vi "Velociprobe_Nanopositioner_Control_RT 2.vi"() -> ()   [LabVIEW 2015]
uses:
  <vilib>/rvi/interface/nirviReadWriteControl/nirviReadWriteControl.xnode
  <vilib>/rvi/interface/Simulation/niFpgaSimulationCallBeginRW.vi
  <vilib>/rvi/errors/niLvFpgaAdjustHostInterfaceError.vi
  <vilib>/rvi/interface/nirviCloseFPGA/nirviCloseFPGA.xnode
  <vilib>/rvi/interface/nirviMethod/nirviMethod.xnode
  <vilib>/rvi/errors/niLvFpgaMergeErrorWithErrorCode.vi
  <vilib>/Platform/TimedLoop/XDataNode/XDataNode.xnode
  <vilib>/Platform/TimedLoop/XDataNode/nitl_modes.ctl
  <vilib>/Platform/TimedLoop/XDataNode/XDNodeRunTimeDep.lvlib
  <vilib>/Platform/TimedLoop/XDataNode/wakeup.ctl
  <vilib>/Platform/TimedLoop/XDataNode/timing_clust.ctl
  <vilib>/rvi/interface/nirviOpenFPGA/nirviOpenFPGA.xnode
  <vilib>/rvi/Analysis/host/Public/NI_FpgaMspHost.lvlib
  State Enum.ctl
  Data Write Control.ctl
  <vilib>/rvi/interface/nirviMethod/StockFPGA_InlinedMethodWaitForSingleIRQ.vi
  <vilib>/FPGAPlugInAG/Dynamic/niLvFpga_WaitOnIrq_Dynamic.vi
  <vilib>/FPGAPlugInAG/Dynamic/niLvFpga_AcknowledgeIrq_Dynamic.vi
  <vilib>/Utility/file.llb/Read Delimited Spreadsheet (DBL).vi
  <vilib>/FPGAPlugInAG/Dynamic/niLvFpga_ConfigureFifo_Dynamic.vi
  NiFpgaLv.dll
  <vilib>/Utility/error.llb/Error Cluster From Error Code.vi
  <vilib>/FPGAPlugInAG/Dynamic/niLvFpga_ReadFifo_Dynamic.vi
  <vilib>/FPGAPlugInAG/Dynamic/niLvFpga_StopFifo_Dynamic.vi
  <vilib>/FPGAPlugInAG/Dynamic/niLvFpga_Close_Dynamic.vi
  FPGA Bitfiles/VelociprobeMIMOC_FPGATarget_VelociprobeNanop_-KB3D2agfK0.lvbitx
  FPGA VIs/Velociprobe_Nanopositioner_Control_FPGA.vi
  <vilib>/FPGAPlugInAG/cRIO-9039/niLvFpga_Open_cRIO-9039.vi
  <vilib>/rvi/interface/common/dynamic/niFpgaDynamicAddResources.vi
panel:
  in  "Tab Control":T1(tab)
  in  "Controller Time Period (uSec)":u32=40
  in  "Controller Output Time Period (uSec)":u32=40
  in  "X Reference Time Period (uSec)":u32=40
  in  "Plant Output Time Period (uSec)":u32=40
  in  "Stop":bool
  in  "Datalog Time Period (uSec)":u32=40
  in  "Analog Input Time Period (uSec)":u32=40
  in  "Detector Trigger Time Period (uSec)":u32=40
  in  "Trigger Generation Time Period (uSec)":u32=40
  in  "Y Reference Time Period (uSec)":u32=40
  in  "Z Reference Time Period (uSec)":u32=40
  in  "Data Trigger Time Period (uSec)":u32=40
  out "Iteration Duration RT Timed-Loop":i64=128
  in  "X Ramp Start (nm)":fxp<+/-,16,16>=-4500.0
  in  "X Ramp End (nm)":fxp<+/-,16,16>=4500.0
  in  "X Start Marker (nm)":fxp<+/-,58,25>
  in  "Y Ramp Start (nm)":fxp<+/-,16,16>=4500.0
  in  "Y Ramp End (nm)":fxp<+/-,16,16>=-4500.0
  in  "Y Vertical Step Size (nm)":fxp<+/-,16,16>=50.0
  in  "Y Start Marker (nm)":fxp<+/-,58,25>
  out "Fly Scan Running":bool
  out "Continue Run":bool
  out "X Ramp Period (usec)":fxp<+,24,24>=60000.0
  out "Y Ramp Period (usec)":fxp<+,24,24>=60000.0
  out "# of Hor Lines":fxp<+/-,34,18>=181.0 format="%.22g"
  in  "X Horizontal Step Size (nm)":fxp<+/-,16,16>=50.0
  out "# of Points per Line":fxp<+/-,33,17>=180.0
  out "# Total Trigger Points":fxp<+/-,64,34>=32580.0
  out "sec per line":dbl=0.06
  out "line per sec (Hz)":dbl=16.666666666666668
  out "X Ramp Period DBL (usec)":dbl=60000.0 format="%#_6f"
  out "Total Scan Time (sec)":dbl=10.86
  in  "Snake Scan Reference FPGA or EPICS":enum16{"FPGA Snake Scan", "EPICS Snake Scan"}(ring)
  in  "Detector Trigger Lower Limit (V)":fxp<+/-,20,5>
  in  "Detector Trigger Upper Limit (V)":fxp<+/-,20,5>=5.0
  out "Detector Trigger (V)":fxp<+/-,20,5>
  out "Detector Trigger In Range?":bool=TRUE
  in  "Trigger High Period (usec)":fxp<+/-,64,45>=1250.0
  in  "Trigger Low Period (usec)":fxp<+/-,64,45>=1250.0
  in  "Trigger High Level (V)":fxp<+/-,20,5>=5.0
  in  "Trigger Low Level (V)":fxp<+/-,20,5>
  in  "Trigger Wave Generator":T2(ring)=enum."Square Wave 1"
  in  "DT Reference Amplitude (V)":fxp<+/-,40,17>=5.0
  in  "DT Reference DC Offset (V)":fxp<+/-,16,16>
  out "DT Frequency (periods/tick)":fxp<+,32,0>=7.500010542571545e-05
  out "DT Phase Offset (periods)":fxp<+,32,0>
  in  "DT Reset":bool
  out "DT Duty Cycle (periods)":fxp<+,32,0>=0.8799999998882413
  in  "DT phase offset (deg)":dbl format="%#.6g"
  in  "DT Frequency (Hz)":dbl=3000.0 format="%#_6p"
  in  "DT duty cycle (%)":dbl=88.0 min=0.0 max=100.0 step=1.0
  in  "name":string="Velociprobe_Id_A344_.csv"
  in  "Write Data":bool
  in  "System Loop Type":enum16{"Open Loop", "Closed Loop"}(ring)=enum."Closed Loop"
  in  "Reset All":bool
  in  "Fly Scan Start":bool
  in  "Z White Noise Seed":u32=4
  in  "Z White Noise Amplitude":u16=32767
  in  "Y White Noise Seed":u32=4
  in  "Y White Noise Amplitude":u16=32767
  in  "Z Reference Reset":bool
  in  "Y Reference Reset":bool
  in  "X Reference Reset":bool
  in  "Z Reference Wave Selection":T3(ring)=enum."Sine Wave"
  in  "X Reference Wave Selection":T4(ring)=enum."Custom Up Down Ramp"
  in  "Y Reference Wave Selection":T5(ring)=enum."Custom Ramp Wave"
  in  "Optics and or Sample Stage":T6(ring)
  out "Z phase offset (periods)":fxp<+,32,0>
  out "Z frequency (periods/tick)":fxp<+,32,0>=1.25030055642128e-07 format="%.32g"
  in  "Z phase offset (deg)":dbl format="%#.6g"
  in  "Z frequency (Hz)":dbl=5.0 format="%#_6p"
  out "Y phase offset (periods)":fxp<+,32,0>
  out "Y frequency (periods/tick)":fxp<+,32,0>=5.005858838558197e-08 format="%.32g"
  in  "Y phase offset (deg)":dbl format="%#.6g"
  in  "Y frequency (Hz)":dbl=2.0 format="%#_6p"
  in  "Scaling mV to V":fxp<+,33,10>=0.001000046730041504
  out "Z Stage Reference (nm)":fxp<+/-,58,25>
  out "Y Stage Reference (nm)":fxp<+/-,58,25>
  out "X Stage Reference (nm)":fxp<+/-,58,25>
  in  "X White Noise Seed":u32=4
  in  "X White Noise Amplitude":u16=32767
  in  "Z Reference DC Offset (nm)":fxp<+/-,15,15>
  in  "Y Reference DC Offset (nm)":fxp<+/-,16,16>
  in  "X Reference DC Offset (nm)":fxp<+/-,16,16>
  in  "Z Reference Amplitude (nm)":fxp<+/-,40,17>
  in  "Y Reference Amplitude (nm)":fxp<+/-,40,17>=100.0
  in  "X Reference Amplitude (nm)":fxp<+/-,40,17>=100.0
  out "X phase offset (periods)":fxp<+,32,0>
  out "X frequency (periods/tick)":fxp<+,32,0>=1.25030055642128e-07 format="%.32g"
  in  "X phase offset (deg)":dbl format="%#.6g"
  in  "X frequency (Hz)":dbl=5.0 format="%#_6p"
  out "Trigger for Data":fxp<+/-,58,25>=1.0
  in  "Z-Stage Scaling Direction":fxp<+/-,3,3>=-1.0
  in  "Y-Stage Scaling Direction":fxp<+/-,3,3>=-1.0
  in  "Mod 3 AI2 V to nm Scaling":fxp<+,47,18>=1000.0
  in  "Mod 3 AI1 V to nm Scaling":fxp<+,47,18>=1000.0
  out "Mod6/DIO3":bool
  out "Mod5/DIO3":bool
  out "Mod4/DIO3":bool
  in  "Sample Z Stage Resolution (nm)":fxp<+,33,3>=0.5
  in  "Sample Y Stage Resolution (nm)":fxp<+,33,3>=0.5
  in  "Sample X Stage Resolution (nm)":fxp<+,33,3>=0.5
  in  "Optics Z Stage Resolution (nm)":fxp<+,33,3>=0.5
  in  "Optics Y Stage Resolution (nm)":fxp<+,33,3>=0.5
  in  "Optics X Stage Resolution (nm)":fxp<+,33,3>=0.5
  in  "Sample Z Reset":bool
  in  "Sample Y Reset":bool
  in  "Sample X Reset":bool
  out "Data":fxp<+/-,58,25>[](array[numeric])
  in  "Mod 3 AI0 V to nm Scaling":fxp<+,47,18>=1000.0
  in  "Timeout FPGA FIFO1":i32=40000000
  out "FIFO Timed Out":bool
  out "stop case":bool
  in  "IRQ Timeout (ms)":i32=10000
  out "IRQ Timed Out":bool
  in  "Datalog Cases":T7(ring)=enum."Data Log 16"
  out "Mod6/DIO2":bool
  out "Mod6/DIO1":bool
  out "Mod6/DIO0":bool=TRUE
  out "Mod5/DIO2":bool
  out "Mod5/DIO1":bool=TRUE
  out "Mod5/DIO0":bool
  out "Mod4/DIO2":bool=TRUE
  out "Mod4/DIO1":bool
  out "Mod4/DIO0":bool=TRUE
  in  "Optics Z Reset":bool
  in  "Optics Y Reset":bool
  in  "Optics X Reset":bool
  out "FIFO Timed Out?":bool
  in  "FIFO Time Period":dbl=0.01 format="%#_13g"
  out "Number of Elements":u32=1250
  out "Datalog Rate (Hz)":dbl=25000.000000000004
  out "Elements Remaining":u32
  in  "Timeout (ms)":i32=10000
  out "Number of Data Strings":i32=5
  out "Z-Stage Input In Range?":bool=TRUE
  out "Y-Stage Input In Range?":bool=TRUE
  out "X-Stage Input In Range?":bool=TRUE
  out "PI Z-Stage Input (V)":fxp<+/-,20,5>=-0.000732421875
  out "PI Y-Stage Input (V)":fxp<+/-,20,5>=0.005584716796875
  out "PI X-Stage Input (V)":fxp<+/-,20,5>=-0.00311279296875
  in  "Z-Stage nm to V Scaling":fxp<+/-,32,12>=0.0005397796630859375
  in  "Y-Stage nm to V Scaling":fxp<+/-,32,12>=0.0014200210571289062
  in  "X-Stage Scaling Direction":fxp<+/-,3,3>=-1.0
  in  "X-Stage nm to V Scaling":fxp<+/-,32,12>=0.0005359649658203125
  in  "Controller Output Lower Limit":fxp<+/-,20,5>=-5.0
  in  "Controller Output Upper Limit":fxp<+/-,20,5>=5.0
  out "Actual Depth":u32=131068416
  in  "Requested Depth":u32=131068000
  out "Waveform Graph 2":cluster{"t0":dbl, dbl, dbl[][]}(graph)={"t0"=0.0, 3.9999999999999996e-05, [[0.0, 0.0, 0.0, 0.0, 0.0, 0.0, 0.0, 0.0, 0.0, 0.0, 0.0, 0.0, 0.0, 0.0, 0.0, 0.0, 0.0, 0.0, 0.0, 0.0, 0.0, 0.0, 0.0, 0.0, 0.0, 0.0, 0.0, 0.0, 0.0, 0.0, 0.0, 0.0, 0.0, 0.0, 0.0, 0.0, 0.0, 0.0, 0.0, 0.0, 0.0, 0.0, 0.0, 0.0, 0.0, 0.0, 0.0, 0.0, 0.0, 0.0, 0.0, 0.0, 0.0, 0.0, 0.0, 0.0, 0.0, 0.0, 0.0, 0.0, 0.0, 0.0, 0.0, 0.0, 0.0, 0.0, 0.0, 0.0, 0.0, 0.0, 0.0, 0.0, 0.0, 0.0, 0.0, 0.0, 0.0, 0.0, 0.0, 0.0, 0.0, 0.0, 0.0, 0.0, 0.0, 0.0, 0.0, 0.0, 0.0, 0.0, 0.0, 0.0, 0.0, 0.0, 0.0, 0.0, 0.0, 0.0, 0.0, 0.0, 0.0, 0.0, 0.0, 0.0, 0.0, 0.0, 0.0, 0.0, 0.0, 0.0, 0.0, 0.0, 0.0, 0.0, 0.0, 0.0, 0.0, 0.0, 0.0, 0.0, 0.0, 0.0, 0.0, 0.0, 0.0, 0.0, 0.0, 0.0, 0.0, 0.0, 0.0, 0.0, 0.0, 0.0, 0.0, 0.0, 0.0, 0.0, 0.0, 0.0, 0.0, 0.0, 0.0, 0.0, 0.0, 0.0, 0.0, 0.0, 0.0, 0.0, 0.0, 0.0, 0.0, 0.0, 0.0, 0.0, 0.0, 0.0, 0.0, 0.0, 0.0, 0.0, 0.0, 0.0, 0.0, 0.0, 0.0, 0.0, 0.0, 0.0, 0.0, 0.0, 0.0, 0.0, 0.0, 0.0, 0.0, 0.0, 0.0, 0.0, 0.0, 0.0, 0.0, 0.0, 0.0, 0.0, 0.0, 0.0, 0.0, 0.0, 0.0, 0.0, 0.0, 0.0, 0.0, 0.0, 0.0, 0.0, 0.0, 0.0, 0.0, 0.0, 0.0, 0.0, 0.0, 0.0, 0.0, 0.0, 0.0, 0.0, 0.0, 0.0, 0.0, 0.0, 0.0, 0.0, 0.0, 0.0, 0.0, 0.0, 0.0, 0.0, 0.0, 0.0, 0.0, 0.0, 0.0, 0.0, 0.0, 0.0, 0.0, 0.0, 0.0, 0.0, 0.0, 0.0, 0.0, 0.0, 0.0, 0.0, 0.0, 0.0, 0.0, 0.0, 0.0, 0.0, 0.0, 0.0, 0.0, 0.0], [0.0, 0.0, 0.0, 0.0, 0.0, 0.0, 0.0, 0.0, 0.0, 0.0, 0.0, 0.0, 0.0, 0.0, 0.0, 0.0, 0.0, 0.0, 0.0, 0.0, 0.0, 0.0, 0.0, 0.0, 0.0, 0.0, 0.0, 0.0, 0.0, 0.0, 0.0, 0.0, 0.0, 0.0, 0.0, 0.0, 0.0, 0.0, 0.0, 0.0, 0.0, 0.0, 0.0, 0.0, 0.0, 0.0, 0.0, 0.0, 0.0, 0.0, 0.0, 0.0, 0.0, 0.0, 0.0, 0.0, 0.0, 0.0, 0.0, 0.0, 0.0, 0.0, 0.0, 0.0, 0.0, 0.0, 0.0, 0.0, 0.0, 0.0, 0.0, 0.0, 0.0, 0.0, 0.0, 0.0, 0.0, 0.0, 0.0, 0.0, 0.0, 0.0, 0.0, 0.0, 0.0, 0.0, 0.0, 0.0, 0.0, 0.0, 0.0, 0.0, 0.0, 0.0, 0.0, 0.0, 0.0, 0.0, 0.0, 0.0, 0.0, 0.0, 0.0, 0.0, 0.0, 0.0, 0.0, 0.0, 0.0, 0.0, 0.0, 0.0, 0.0, 0.0, 0.0, 0.0, 0.0, 0.0, 0.0, 0.0, 0.0, 0.0, 0.0, 0.0, 0.0, 0.0, 0.0, 0.0, 0.0, 0.0, 0.0, 0.0, 0.0, 0.0, 0.0, 0.0, 0.0, 0.0, 0.0, 0.0, 0.0, 0.0, 0.0, 0.0, 0.0, 0.0, 0.0, 0.0, 0.0, 0.0, 0.0, 0.0, 0.0, 0.0, 0.0, 0.0, 0.0, 0.0, 0.0, 0.0, 0.0, 0.0, 0.0, 0.0, 0.0, 0.0, 0.0, 0.0, 0.0, 0.0, 0.0, 0.0, 0.0, 0.0, 0.0, 0.0, 0.0, 0.0, 0.0, 0.0, 0.0, 0.0, 0.0, 0.0, 0.0, 0.0, 0.0, 0.0, 0.0, 0.0, 0.0, 0.0, 0.0, 0.0, 0.0, 0.0, 0.0, 0.0, 0.0, 0.0, 0.0, 0.0, 0.0, 0.0, 0.0, 0.0, 0.0, 0.0, 0.0, 0.0, 0.0, 0.0, 0.0, 0.0, 0.0, 0.0, 0.0, 0.0, 0.0, 0.0, 0.0, 0.0, 0.0, 0.0, 0.0, 0.0, 0.0, 0.0, 0.0, 0.0, 0.0, 0.0, 0.0, 0.0, 0.0, 0.0, 0.0, 0.0, 0.0, 0.0, 0.0, 0.0, 0.0, 0.0, 0.0, 0.0, 0.0, 0.0, 0.0, 0.0], [0.0, 0.0, 0.0, 0.0, 0.0, 0.0, 0.0, 0.0, 0.0, 0.0, 0.0, 0.0, 0.0, 0.0, 0.0, 0.0, 0.0, 0.0, 0.0, 0.0, 0.0, 0.0, 0.0, 0.0, 0.0, 0.0, 0.0, 0.0, 0.0, 0.0, 0.0, 0.0, 0.0, 0.0, 0.0, 0.0, 0.0, 0.0, 0.0, 0.0, 0.0, 0.0, 0.0, 0.0, 0.0, 0.0, 0.0, 0.0, 0.0, 0.0, 0.0, 0.0, 0.0, 0.0, 0.0, 0.0, 0.0, 0.0, 0.0, 0.0, 0.0, 0.0, 0.0, 0.0, 0.0, 0.0, 0.0, 0.0, 0.0, 0.0, 0.0, 0.0, 0.0, 0.0, 0.0, 0.0, 0.0, 0.0, 0.0, 0.0, 0.0, 0.0, 0.0, 0.0, 0.0, 0.0, 0.0, 0.0, 0.0, 0.0, 0.0, 0.0, 0.0, 0.0, 0.0, 0.0, 0.0, 0.0, 0.0, 0.0, 0.0, 0.0, 0.0, 0.0, 0.0, 0.0, 0.0, 0.0, 0.0, 0.0, 0.0, 0.0, 0.0, 0.0, 0.0, 0.0, 0.0, 0.0, 0.0, 0.0, 0.0, 0.0, 0.0, 0.0, 0.0, 0.0, 0.0, 0.0, 0.0, 0.0, 0.0, 0.0, 0.0, 0.0, 0.0, 0.0, 0.0, 0.0, 0.0, 0.0, 0.0, 0.0, 0.0, 0.0, 0.0, 0.0, 0.0, 0.0, 0.0, 0.0, 0.0, 0.0, 0.0, 0.0, 0.0, 0.0, 0.0, 0.0, 0.0, 0.0, 0.0, 0.0, 0.0, 0.0, 0.0, 0.0, 0.0, 0.0, 0.0, 0.0, 0.0, 0.0, 0.0, 0.0, 0.0, 0.0, 0.0, 0.0, 0.0, 0.0, 0.0, 0.0, 0.0, 0.0, 0.0, 0.0, 0.0, 0.0, 0.0, 0.0, 0.0, 0.0, 0.0, 0.0, 0.0, 0.0, 0.0, 0.0, 0.0, 0.0, 0.0, 0.0, 0.0, 0.0, 0.0, 0.0, 0.0, 0.0, 0.0, 0.0, 0.0, 0.0, 0.0, 0.0, 0.0, 0.0, 0.0, 0.0, 0.0, 0.0, 0.0, 0.0, 0.0, 0.0, 0.0, 0.0, 0.0, 0.0, 0.0, 0.0, 0.0, 0.0, 0.0, 0.0, 0.0, 0.0, 0.0, 0.0, 0.0, 0.0, 0.0, 0.0, 0.0, 0.0, 0.0, 0.0, 0.0, 0.0, 0.0, 0.0], [0.0, 0.0, 0.0, 0.0, 0.0, 0.0, 0.0, 0.0, 0.0, 0.0, 0.0, 0.0, 0.0, 0.0, 0.0, 0.0, 0.0, 0.0, 0.0, 0.0, 0.0, 0.0, 0.0, 0.0, 0.0, 0.0, 0.0, 0.0, 0.0, 0.0, 0.0, 0.0, 0.0, 0.0, 0.0, 0.0, 0.0, 0.0, 0.0, 0.0, 0.0, 0.0, 0.0, 0.0, 0.0, 0.0, 0.0, 0.0, 0.0, 0.0, 0.0, 0.0, 0.0, 0.0, 0.0, 0.0, 0.0, 0.0, 0.0, 0.0, 0.0, 0.0, 0.0, 0.0, 0.0, 0.0, 0.0, 0.0, 0.0, 0.0, 0.0, 0.0, 0.0, 0.0, 0.0, 0.0, 0.0, 0.0, 0.0, 0.0, 0.0, 0.0, 0.0, 0.0, 0.0, 0.0, 0.0, 0.0, 0.0, 0.0, 0.0, 0.0, 0.0, 0.0, 0.0, 0.0, 0.0, 0.0, 0.0, 0.0, 0.0, 0.0, 0.0, 0.0, 0.0, 0.0, 0.0, 0.0, 0.0, 0.0, 0.0, 0.0, 0.0, 0.0, 0.0, 0.0, 0.0, 0.0, 0.0, 0.0, 0.0, 0.0, 0.0, 0.0, 0.0, 0.0, 0.0, 0.0, 0.0, 0.0, 0.0, 0.0, 0.0, 0.0, 0.0, 0.0, 0.0, 0.0, 0.0, 0.0, 0.0, 0.0, 0.0, 0.0, 0.0, 0.0, 0.0, 0.0, 0.0, 0.0, 0.0, 0.0, 0.0, 0.0, 0.0, 0.0, 0.0, 0.0, 0.0, 0.0, 0.0, 0.0, 0.0, 0.0, 0.0, 0.0, 0.0, 0.0, 0.0, 0.0, 0.0, 0.0, 0.0, 0.0, 0.0, 0.0, 0.0, 0.0, 0.0, 0.0, 0.0, 0.0, 0.0, 0.0, 0.0, 0.0, 0.0, 0.0, 0.0, 0.0, 0.0, 0.0, 0.0, 0.0, 0.0, 0.0, 0.0, 0.0, 0.0, 0.0, 0.0, 0.0, 0.0, 0.0, 0.0, 0.0, 0.0, 0.0, 0.0, 0.0, 0.0, 0.0, 0.0, 0.0, 0.0, 0.0, 0.0, 0.0, 0.0, 0.0, 0.0, 0.0, 0.0, 0.0, 0.0, 0.0, 0.0, 0.0, 0.0, 0.0, 0.0, 0.0, 0.0, 0.0, 0.0, 0.0, 0.0, 0.0, 0.0, 0.0, 0.0, 0.0, 0.0, 0.0, 0.0, 0.0, 0.0, 0.0, 0.0, 0.0], [0.0, 0.0, 0.0, 0.0, 0.0, 0.0, 0.0, 0.0, 0.0, 0.0, 0.0, 0.0, 0.0, 0.0, 0.0, 0.0, 0.0, 0.0, 0.0, 0.0, 0.0, 0.0, 0.0, 0.0, 0.0, 0.0, 0.0, 0.0, 0.0, 0.0, 0.0, 0.0, 0.0, 0.0, 0.0, 0.0, 0.0, 0.0, 0.0, 0.0, 0.0, 0.0, 0.0, 0.0, 0.0, 0.0, 0.0, 0.0, 0.0, 0.0, 0.0, 0.0, 0.0, 0.0, 0.0, 0.0, 0.0, 0.0, 0.0, 0.0, 0.0, 0.0, 0.0, 0.0, 0.0, 0.0, 0.0, 0.0, 0.0, 0.0, 0.0, 0.0, 0.0, 0.0, 0.0, 0.0, 0.0, 0.0, 0.0, 0.0, 0.0, 0.0, 0.0, 0.0, 0.0, 0.0, 0.0, 0.0, 0.0, 0.0, 0.0, 0.0, 0.0, 0.0, 0.0, 0.0, 0.0, 0.0, 0.0, 0.0, 0.0, 0.0, 0.0, 0.0, 0.0, 0.0, 0.0, 0.0, 0.0, 0.0, 0.0, 0.0, 0.0, 0.0, 0.0, 0.0, 0.0, 0.0, 0.0, 0.0, 0.0, 0.0, 0.0, 0.0, 0.0, 0.0, 0.0, 0.0, 0.0, 0.0, 0.0, 0.0, 0.0, 0.0, 0.0, 0.0, 0.0, 0.0, 0.0, 0.0, 0.0, 0.0, 0.0, 0.0, 0.0, 0.0, 0.0, 0.0, 0.0, 0.0, 0.0, 0.0, 0.0, 0.0, 0.0, 0.0, 0.0, 0.0, 0.0, 0.0, 0.0, 0.0, 0.0, 0.0, 0.0, 0.0, 0.0, 0.0, 0.0, 0.0, 0.0, 0.0, 0.0, 0.0, 0.0, 0.0, 0.0, 0.0, 0.0, 0.0, 0.0, 0.0, 0.0, 0.0, 0.0, 0.0, 0.0, 0.0, 0.0, 0.0, 0.0, 0.0, 0.0, 0.0, 0.0, 0.0, 0.0, 0.0, 0.0, 0.0, 0.0, 0.0, 0.0, 0.0, 0.0, 0.0, 0.0, 0.0, 0.0, 0.0, 0.0, 0.0, 0.0, 0.0, 0.0, 0.0, 0.0, 0.0, 0.0, 0.0, 0.0, 0.0, 0.0, 0.0, 0.0, 0.0, 0.0, 0.0, 0.0, 0.0, 0.0, 0.0, 0.0, 0.0, 0.0, 0.0, 0.0, 0.0, 0.0, 0.0, 0.0, 0.0, 0.0, 0.0, 0.0, 0.0, 0.0, 0.0, 0.0, 0.0]]}
  out "Elements Remaining Waveform Chart":u32(graph)
  out "Elements Remaining Waveform Chart 3":u32(graph)
  out "XY Graph":cluster{"Array":dbl[], "Array":dbl[]}(graph)
  out "XY Graph 2":cluster{"Array":dbl[], "Array":dbl[]}(graph)
  out "Measured Datalog Time Period (Ticks)":u32=1600
  out "Measured Datalog Loop Rate (secs)":dbl=3.9999999999999996e-05
  out "Measured Datalog Loop Rate (kHz)":dbl=25.000000000000004
  out "Measured Counter Loop Rate (secs)":dbl
  out "Measured Counter Loop Rate (MHz)":dbl=inf
  out "Measured X Reference Loop Rate (secs)":dbl=3.9999999999999996e-05
  out "Measured X Reference Loop Rate (kHz)":dbl=25.000000000000004
  out "Measured X Reference Time Period (Ticks)":u32=1600
  out "Measured Controller Loop Rate (kHz)":dbl=25.000000000000004
  out "Measured Controller Output Loop Rate (secs)":dbl=3.9999999999999996e-05
  out "Measured Controller Output Loop Rate (kHz)":dbl=25.000000000000004
  out "Measured Plant Output Loop Rate (secs)":dbl=3.9999999999999996e-05
  out "Measured Plant Output Loop Rate (kHz)":dbl=25.000000000000004
  out "Measured Controller Loop Rate (secs)":dbl=3.9999999999999996e-05
  out "Measured Controller Time Period (Ticks)":u32=1600
  out "Datalog Time Period (sec)":dbl=3.9999999999999996e-05
  out "Measured Controller Output Time Period (Ticks)":u32=1600
  out "Measured Plant Output Time Period (Ticks)":u32=1600
  out "Measured Counter Time Period (Ticks)":u32
  out "32 bit Count Optics X":i32
  out "32 bit Count Optics  Y":i32
  out "32 bit Count Optics  Z":i32
  out "32 bit Count Sample X":i32
  out "32 bit Count Sample  Y":i32=2
  out "32 bit Count Sample  Z":i32=-4
  out "Optics X Stage Displacement (nm)":fxp<+/-,58,25>=-1.0
  out "Optics Y Stage Displacement (nm)":fxp<+/-,58,25>
  out "Optics Z Stage Displacement (nm)":fxp<+/-,58,25>
  out "Sample X Stage Displacement (nm)":fxp<+/-,58,25>=-0.5
  out "Sample Y Stage Displacement (nm)":fxp<+/-,58,25>=1.5
  out "Sample Z Stage Displacement (nm)":fxp<+/-,58,25>=-1.0
  out "Measured Analog Input Time Period (Ticks)":u32=1600
  out "Measured Analog Input Loop Rate (secs)":dbl=3.9999999999999996e-05
  out "Measured Analog Input Loop Rate (kHz)":dbl=25.000000000000004
  out "Measured Detector Trigger Time Period (Ticks)":u32=1600
  out "Measured Trigger Gen Time Period (Ticks)":u32=1600
  out "Measured Y Reference Time Period (Ticks)":u32=1600
  out "Measured Z Reference Time Period (Ticks)":u32=1600
  out "Measured Y Reference Loop Rate (secs)":dbl=3.9999999999999996e-05
  out "Measured Y Reference Loop Rate (kHz)":dbl=25.000000000000004
  out "Measured Z Reference Loop Rate (secs)":dbl=3.9999999999999996e-05
  out "Measured Z Reference Loop Rate (kHz)":dbl=25.000000000000004
  out "Measured Data Trigger Time Period (Ticks)":u32=1600
  out "message":string="No Error"
  out "2iddVELO:VP:X_End_nm":dbl=2000.0
  out "2iddVELO:VP:X_Start_nm":dbl=-2000.0
  out "2iddVELO:VP:Flyscan_Start":bool
  out "2iddVELO:VP:Y_Start_nm":dbl=2000.0
  out "2iddVELO:VP:Y_End_nm":dbl=-2000.0
  out "2iddVELO:VP:Y_Step_Size_nm":dbl=50.0
  out "2iddVELO:VP:X_Step_Size_nm":dbl=50.0
  out "2iddVELO:VP:Trigger_Freq_Hz":dbl=1000.0
  out "2iddVELO:VP:Write_Data":bool
  out "2iddVELO:VP:Trig_DutyCycle_Per":dbl=99.0
  in  "file path soscoeff_xx1":path=path "C:/ni-rt/startup/2 ID D/Kxx/Kxx_1_Gxx_md_40us/Kxx_1_Gxx_matched_dow_16ord_mVpnm_cd8a3_AvTio9_X5nm_500pm_all_40us_soscof_xx1.mat"
  in  "file path sos gain SF Controller_xx1":path=path "C:/ni-rt/startup/2 ID D/Kxx/Kxx_1_Gxx_md_40us/Kxx_1_Gxx_matched_dow_16ord_mVpnm_cd8a3_AvTio9_X5nm_500pm_all_40us_soscof_xx2.mat"
  in  "file path soscoeff_yy1":path=path "C:/ni-rt/startup/2 ID D/Kyy/Kyy_trial_1_Gyy_md_40us/Kyy_trial_1_Gyy_matched_dow_8ord_mVpnm_cd8a3_AvTio9_Y5nm_500pm_all_40us_soscof_yy1.mat"
  in  "file path sos gain SF Controller_yy1":path=path "C:/ni-rt/startup/2 ID D/Kyy/Kyy_trial_1_Gyy_md_40us/Kyy_trial_1_Gyy_matched_dow_8ord_mVpnm_cd8a3_AvTio9_Y5nm_500pm_all_40us_soscof_yy2.mat"
  in  "file path soscoeff_zz1":path=path "C:/ni-rt/startup/2 ID D/Kzz/Kzz_1_Gzz_md_40us/Kzz_1_Gzz_matched_dow_29ord_mVpnm_cd8a3_AvTio9_Z5nm_500pm_all_40us_soscof_zz1.mat"
  in  "file path sos gain SF Controller_zz1":path=path "C:/ni-rt/startup/2 ID D/Kzz/Kzz_1_Gzz_md_40us/Kzz_1_Gzz_matched_dow_29ord_mVpnm_cd8a3_AvTio9_Z5nm_500pm_all_40us_soscof_zz2.mat"
  in  "file path soscoeff_yx1":path=path "C:/ni-rt/startup/2 ID D/Kxx/Kxx_1_Gxx_md_40us/allzero_mVpnm_XX_XY_XZ_YX_YY_YZ_ZX_ZY_ZZ_woffst_soscoeff1.mat"
  in  "file path sos gain SF Controller_yx1":path=path "C:/ni-rt/startup/2 ID D/Kxx/Kxx_1_Gxx_md_40us/allzero_mVpnm_XX_XY_XZ_YX_YY_YZ_ZX_ZY_ZZ_woffst_soscoeff2.mat"
  in  "file path soscoeff_zx1":path=path "C:/ni-rt/startup/2 ID D/Kxx/Kxx_1_Gxx_md_40us/allzero_mVpnm_XX_XY_XZ_YX_YY_YZ_ZX_ZY_ZZ_woffst_soscoeff1.mat"
  in  "file path sos gain SF Controller_zx1":path=path "C:/ni-rt/startup/2 ID D/Kxx/Kxx_1_Gxx_md_40us/allzero_mVpnm_XX_XY_XZ_YX_YY_YZ_ZX_ZY_ZZ_woffst_soscoeff2.mat"
  in  "file path soscoeff_xy1":path=path "C:/ni-rt/startup/2 ID D/Kxx/Kxx_1_Gxx_md_40us/allzero_mVpnm_XX_XY_XZ_YX_YY_YZ_ZX_ZY_ZZ_woffst_soscoeff1.mat"
  in  "file path sos gain SF Controller_xy1":path=path "C:/ni-rt/startup/2 ID D/Kxx/Kxx_1_Gxx_md_40us/allzero_mVpnm_XX_XY_XZ_YX_YY_YZ_ZX_ZY_ZZ_woffst_soscoeff2.mat"
  in  "file path soscoeff_zy1":path=path "C:/ni-rt/startup/2 ID D/Kxx/Kxx_1_Gxx_md_40us/allzero_mVpnm_XX_XY_XZ_YX_YY_YZ_ZX_ZY_ZZ_woffst_soscoeff1.mat"
  in  "file path sos gain SF Controller_zy1":path=path "C:/ni-rt/startup/2 ID D/Kxx/Kxx_1_Gxx_md_40us/allzero_mVpnm_XX_XY_XZ_YX_YY_YZ_ZX_ZY_ZZ_woffst_soscoeff2.mat"
  in  "file path soscoeff_xz1":path=path "C:/ni-rt/startup/2 ID D/Kxx/Kxx_1_Gxx_md_40us/allzero_mVpnm_XX_XY_XZ_YX_YY_YZ_ZX_ZY_ZZ_woffst_soscoeff1.mat"
  in  "file path sos gain SF Controller_xz1":path=path "C:/ni-rt/startup/2 ID D/Kxx/Kxx_1_Gxx_md_40us/allzero_mVpnm_XX_XY_XZ_YX_YY_YZ_ZX_ZY_ZZ_woffst_soscoeff2.mat"
  in  "file path soscoeff_yz1":path=path "C:/ni-rt/startup/2 ID D/Kxx/Kxx_1_Gxx_md_40us/allzero_mVpnm_XX_XY_XZ_YX_YY_YZ_ZX_ZY_ZZ_woffst_soscoeff1.mat"
  in  "file path sos gain SF Controller_yz1":path=path "C:/ni-rt/startup/2 ID D/Kxx/Kxx_1_Gxx_md_40us/allzero_mVpnm_XX_XY_XZ_YX_YY_YZ_ZX_ZY_ZZ_woffst_soscoeff2.mat"
  out "-a01(2) xx1c":fxp<+/-,64,9>[](array[numeric])=[0.637785025840232, 0.9924182654286198, 1.8461027816316544, 0.8635404845716299, 1.0670555456779864, 1.6350703383821101, 1.6323955588345012, 1.1102241390539636, 0.0, 0.0, 0.0, 0.0, 0.0, 0.0, 0.0, 0.0, 0.0, 0.0, 0.0, 0.0]
  out "-a02(2) xx1c":fxp<+/-,64,9>[](array[numeric])=[-0.999855815746439, -0.9676991072632725, -0.9642268720534838, -0.9446498323360957, -0.9442808087139987, -0.7547983908829242, -0.6690016013017409, -0.11027986125857198, 0.0, 0.0, 0.0, 0.0, 0.0, 0.0, 0.0, 0.0, 0.0, 0.0, 0.0, 0.0]
  out "b01(2) xx1c":fxp<+/-,64,9>[](array[numeric])=[-0.6378105164532328, -1.0062332697665268, -1.8762916543815855, -0.8616288879491845, -1.0856571140792324, -1.6862585929720944, -1.743591709663851, -0.6129835805090948, 0.0, 0.0, 0.0, 0.0, 0.0, 0.0, 0.0, 0.0, 0.0, 0.0, 0.0, 0.0]
  out "b02(2) xx1c":fxp<+/-,64,9>[](array[numeric])=[0.9999102047610771, 0.9971375605901365, 0.9926840301018772, 0.9509648854364836, 0.9563369558920378, 0.7818900462139817, 0.7642575436257291, 3.0531133177191805e-16, 0.0, 0.0, 0.0, 0.0, 0.0, 0.0, 0.0, 0.0, 0.0, 0.0, 0.0, 0.0]
  out "sos gain SF Controller xx1c":fxp<+/-,42,9>=-0.1625035791657865
  out "-a01(2) yy1c":fxp<+/-,64,9>[](array[numeric])=[1.8740229377643998, 1.3096977339382483, 1.7453886241944765, 0.2668895009727739, 0.0, 0.0, 0.0, 0.0, 0.0, 0.0, 0.0, 0.0, 0.0, 0.0, 0.0, 0.0, 0.0, 0.0, 0.0, 0.0]
  out "-a02(2) yy1c":fxp<+/-,64,9>[](array[numeric])=[-0.9732703278433918, -0.5194903821190732, -0.7453924481836136, -2.7755575615628914e-17, 0.0, 0.0, 0.0, 0.0, 0.0, 0.0, 0.0, 0.0, 0.0, 0.0, 0.0, 0.0, 0.0, 0.0, 0.0, 0.0]
  out "b01(2) yy1c":fxp<+/-,64,9>[](array[numeric])=[-1.8979173162254057, -1.8463149313261074, -1.7151162246453355, -0.006444279582847878, 0.0, 0.0, 0.0, 0.0, 0.0, 0.0, 0.0, 0.0, 0.0, 0.0, 0.0, 0.0, 0.0, 0.0, 0.0, 0.0]
  out "b02(2) yy1c":fxp<+/-,64,9>[](array[numeric])=[0.9969084979865663, 0.9421233904433339, 0.7362048104846675, 0.0, 0.0, 0.0, 0.0, 0.0, 0.0, 0.0, 0.0, 0.0, 0.0, 0.0, 0.0, 0.0, 0.0, 0.0, 0.0, 0.0]
  out "sos gain SF Controller yy1c":fxp<+/-,42,9>=-1.480983349494636
  out "-a01(2) zz1c":fxp<+/-,64,9>[](array[numeric])=[0.6242394224317618, 1.8967038692417004, 0.6659160318030806, 1.7792660019034106, 1.6870099721477447, 0.6417945190222861, 1.4838029149808185, 1.8456549628851837, 1.2189509782386598, 0.9933314517253298, 1.0158915520299678, 0.8863484387433826, 0.026837806879254994, 1.8269783715122585, 0.22448441435364225, 0.0, 0.0, 0.0, 0.0, 0.0]
  out "-a02(2) zz1c":fxp<+/-,64,9>[](array[numeric])=[-0.9983298461163967, -0.9972287452752734, -0.995744457243837, -0.9947210838396919, -0.9925914602095722, -0.9920974045271405, -0.9881915357970101, -0.9800069383591395, -0.9760641145386646, -0.9508624135515895, -0.9242774595356998, -0.655945641403593, -0.008661844724279444, -0.8269827070369743, 0.0, 0.0, 0.0, 0.0, 0.0, 0.0]
  out "b01(2) zz1c":fxp<+/-,64,9>[](array[numeric])=[-0.6245671059510156, -1.897930093390194, -0.6670970070931089, -1.7670265604573054, -1.6833314913922348, -0.6327437892303018, -1.5025901530730128, -1.8636454269915796, -1.1210694827766767, -0.9982206064398196, -1.0326369335418408, -1.1342635673267367, -1.6852506306166828, -0.9843740162364313, -1.7208456881689926e-15, 0.0, 0.0, 0.0, 0.0, 0.0]
  out "b02(2) zz1c":fxp<+/-,64,9>[](array[numeric])=[0.9973135069419645, 0.9951302056171929, 0.9993435624612031, 0.9919371251860779, 0.994931751453586, 0.9881092761723503, 0.9884874399279107, 0.9977145546300196, 0.9725302934743221, 0.9855561672767964, 0.9893454712398023, 0.846212786518208, 0.7855598927779743, 0.0978075435519738, 0.0, 0.0, 0.0, 0.0, 0.0, 0.0]
  out "sos gain SF Controller zz1c":fxp<+/-,42,9>=-0.1988595259608701
  out "-a01(2) yx1c":fxp<+/-,64,9>[](array[numeric])
  out "-a02(2) yx1c":fxp<+/-,64,9>[](array[numeric])
  out "b01(2) yx1c":fxp<+/-,64,9>[](array[numeric])
  out "b02(2) yx1c":fxp<+/-,64,9>[](array[numeric])
  out "sos gain SF Controller yx1c":fxp<+/-,42,9>
  out "-a01(2) zx1c":fxp<+/-,64,9>[](array[numeric])
  out "-a02(2) zx1c":fxp<+/-,64,9>[](array[numeric])
  out "b01(2) zx1c":fxp<+/-,64,9>[](array[numeric])
  out "b02(2) zx1c":fxp<+/-,64,9>[](array[numeric])
  out "sos gain SF Controller zx1c":fxp<+/-,42,9>
  out "-a01(2) xy1c":fxp<+/-,64,9>[](array[numeric])
  out "-a02(2) xy1c":fxp<+/-,64,9>[](array[numeric])
  out "b01(2) xy1c":fxp<+/-,64,9>[](array[numeric])
  out "b02(2) xy1c":fxp<+/-,64,9>[](array[numeric])
  out "sos gain SF Controller xy1c":fxp<+/-,42,9>
  out "-a01(2) zy1c":fxp<+/-,64,9>[](array[numeric])
  out "-a02(2) zy1c":fxp<+/-,64,9>[](array[numeric])
  out "b01(2) zy1c":fxp<+/-,64,9>[](array[numeric])
  out "b02(2) zy1c":fxp<+/-,64,9>[](array[numeric])
  out "sos gain SF Controller zy1c":fxp<+/-,42,9>
  out "-a01(2) xz1c":fxp<+/-,64,9>[](array[numeric])
  out "-a02(2) xz1c":fxp<+/-,64,9>[](array[numeric])
  out "b01(2) xz1c":fxp<+/-,64,9>[](array[numeric])
  out "b02(2) xz1c":fxp<+/-,64,9>[](array[numeric])
  out "sos gain SF Controller xz1c":fxp<+/-,42,9>
  out "-a01(2) yz1c":fxp<+/-,64,9>[](array[numeric])
  out "-a02(2) yz1c":fxp<+/-,64,9>[](array[numeric])
  out "b01(2) yz1c":fxp<+/-,64,9>[](array[numeric])
  out "b02(2) yz1c":fxp<+/-,64,9>[](array[numeric])
  out "sos gain SF Controller yz1c":fxp<+/-,42,9>
  out "error out (Sig Gen)":errorcluster
  out "error out (FPGA)":errorcluster
  out "error out (AO FPGA)":errorcluster
  out "Error (RT)":errorcluster
  out "error out (Sig Gen) 2":errorcluster
  out "error out (Sig Gen) 3":errorcluster
  out "error out (Sig Gen) 4":errorcluster
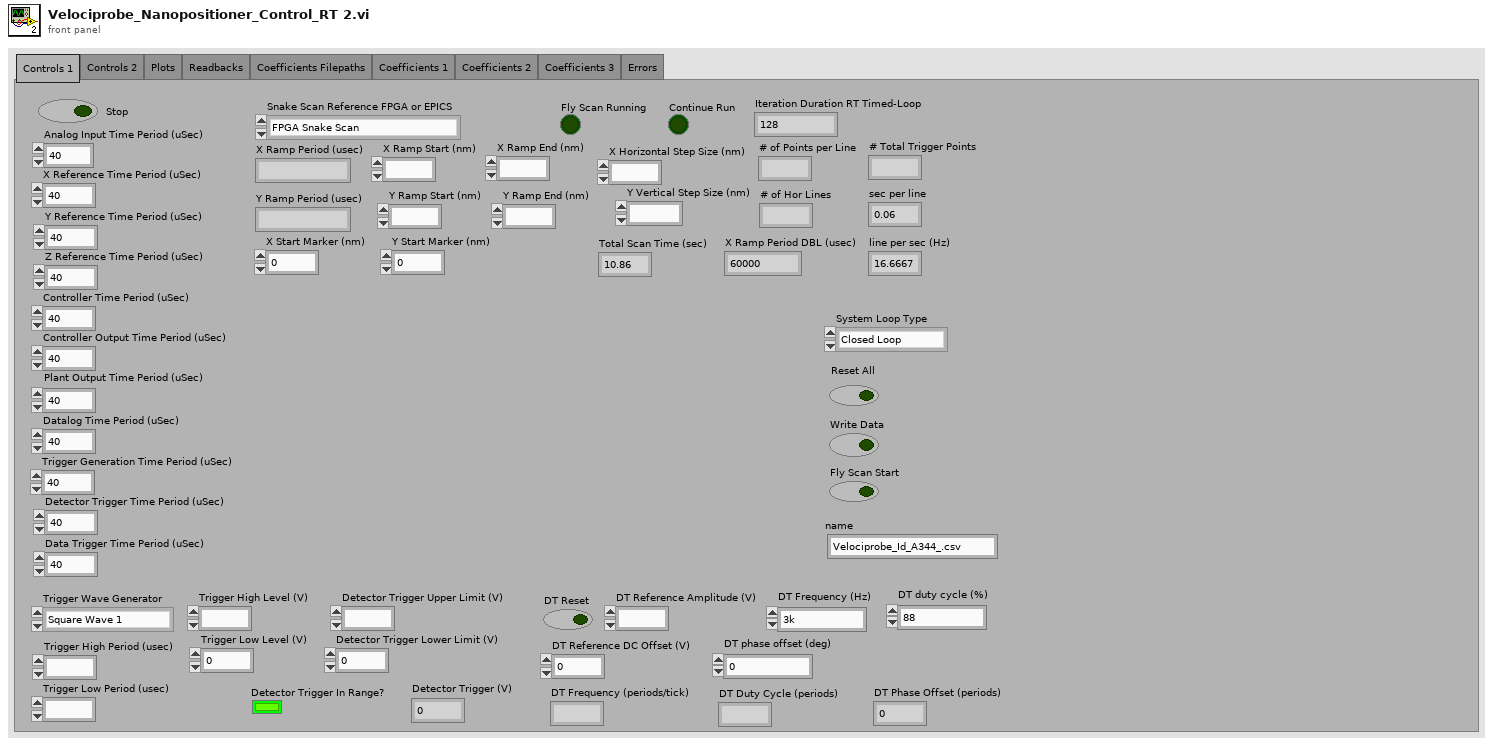
[diagram p1: front panel]
types:
  T1 = enum32{"Controls 1", "Controls 2", "Plots", "Readbacks", "Coefficients Filepaths", "Coefficients 1", "Coefficients 2", "Coefficients 3", "Errors"}
  T2 = enum16{"Custom Square Wave ", "Square Wave 1", "Square Wave 2"}
  T3 = enum16{"Constant", "Sine Wave", "Sawtooth Wave", "Square Wave", "Filtered White Noise"}
  T4 = enum16{"Constant", "Sine Wave", "Custom Up Down Ramp", "Filtered White Noise"}
  T5 = enum16{"Constant", "Sine Wave", "Custom Ramp Wave", "Filtered White Noise"}
  T6 = enum16{"Optics Stage Only", "Optics and Sample Stage"}
  T7 = enum16{"Data Log 1", "Data Log 2", "Data Log 3", "Data Log 4", "Data Log 5", "Data Log 6", "Data Log 7", "Data Log 8", "Data Log 9", "Data Log 10", "Data Log 11", "Data Log 12", "Data Log 13", "Data Log 14", "Data Log 15", "Data Log 16"}
  T8 = typedef "State Enum.ctl" = enum16{"Initialization", "Update Controller Info", "Update Reference Info", "Update Detector Trigger Info", "Update Datalog Info", "Check FPGA Status", "Reading FIFO", "Exit"}
  T9 = typedef "XDNodeRunTimeDep.lvlib/timing_clust.ctl" = cluster{"Expected End [f-1]":u64, "Actual End [f-1]":u64, "Finished Late? [f-1]":bool, "Expected End [i-1]":u64, "Actual End [i-1]":u64, "Finished Late? [i-1]":bool, "Expected Start [i]":u64, "Actual Start [i]":u64, "Expected Start [f]":u64, "Actual Start [f]":u64, "Source Name":string, "Structure Name":string, "Period":i64, "Deadline":i64, "Offset":i64, "Start":i64, "Priority":i32, "Timeout":i32, "Mode":T10, "Wakeup Reason":T11, "Error":errorcluster, "Source Type":string, "Secondary Source Type":string, "Global End Time":u64, "Global Start Time":u64, "Frame Duration":u64, "Iteration Duration":u64, "Assigned CPU":i32, "I/O Scan Engine Mode":u32}
  T10 = typedef "XDNodeRunTimeDep.lvlib/nitl_modes.ctl" = enum32{"No Change", "Process missed periods, maintain original phase", "Discard missed periods, maintain original phase", "Process missed periods, ignore original phase", "Discard missed periods, ignore original phase"}
  T11 = typedef "XDNodeRunTimeDep.lvlib/wakeup.ctl" = enum32{"Normal", "Aborted", "Asynchronous wakeup", "Timing source error", "Timed loop error", "Timeout"}
  T12 = typedef "Data Write Control.ctl" = enum16{"Initialize", "Read", "Write", "Close"}
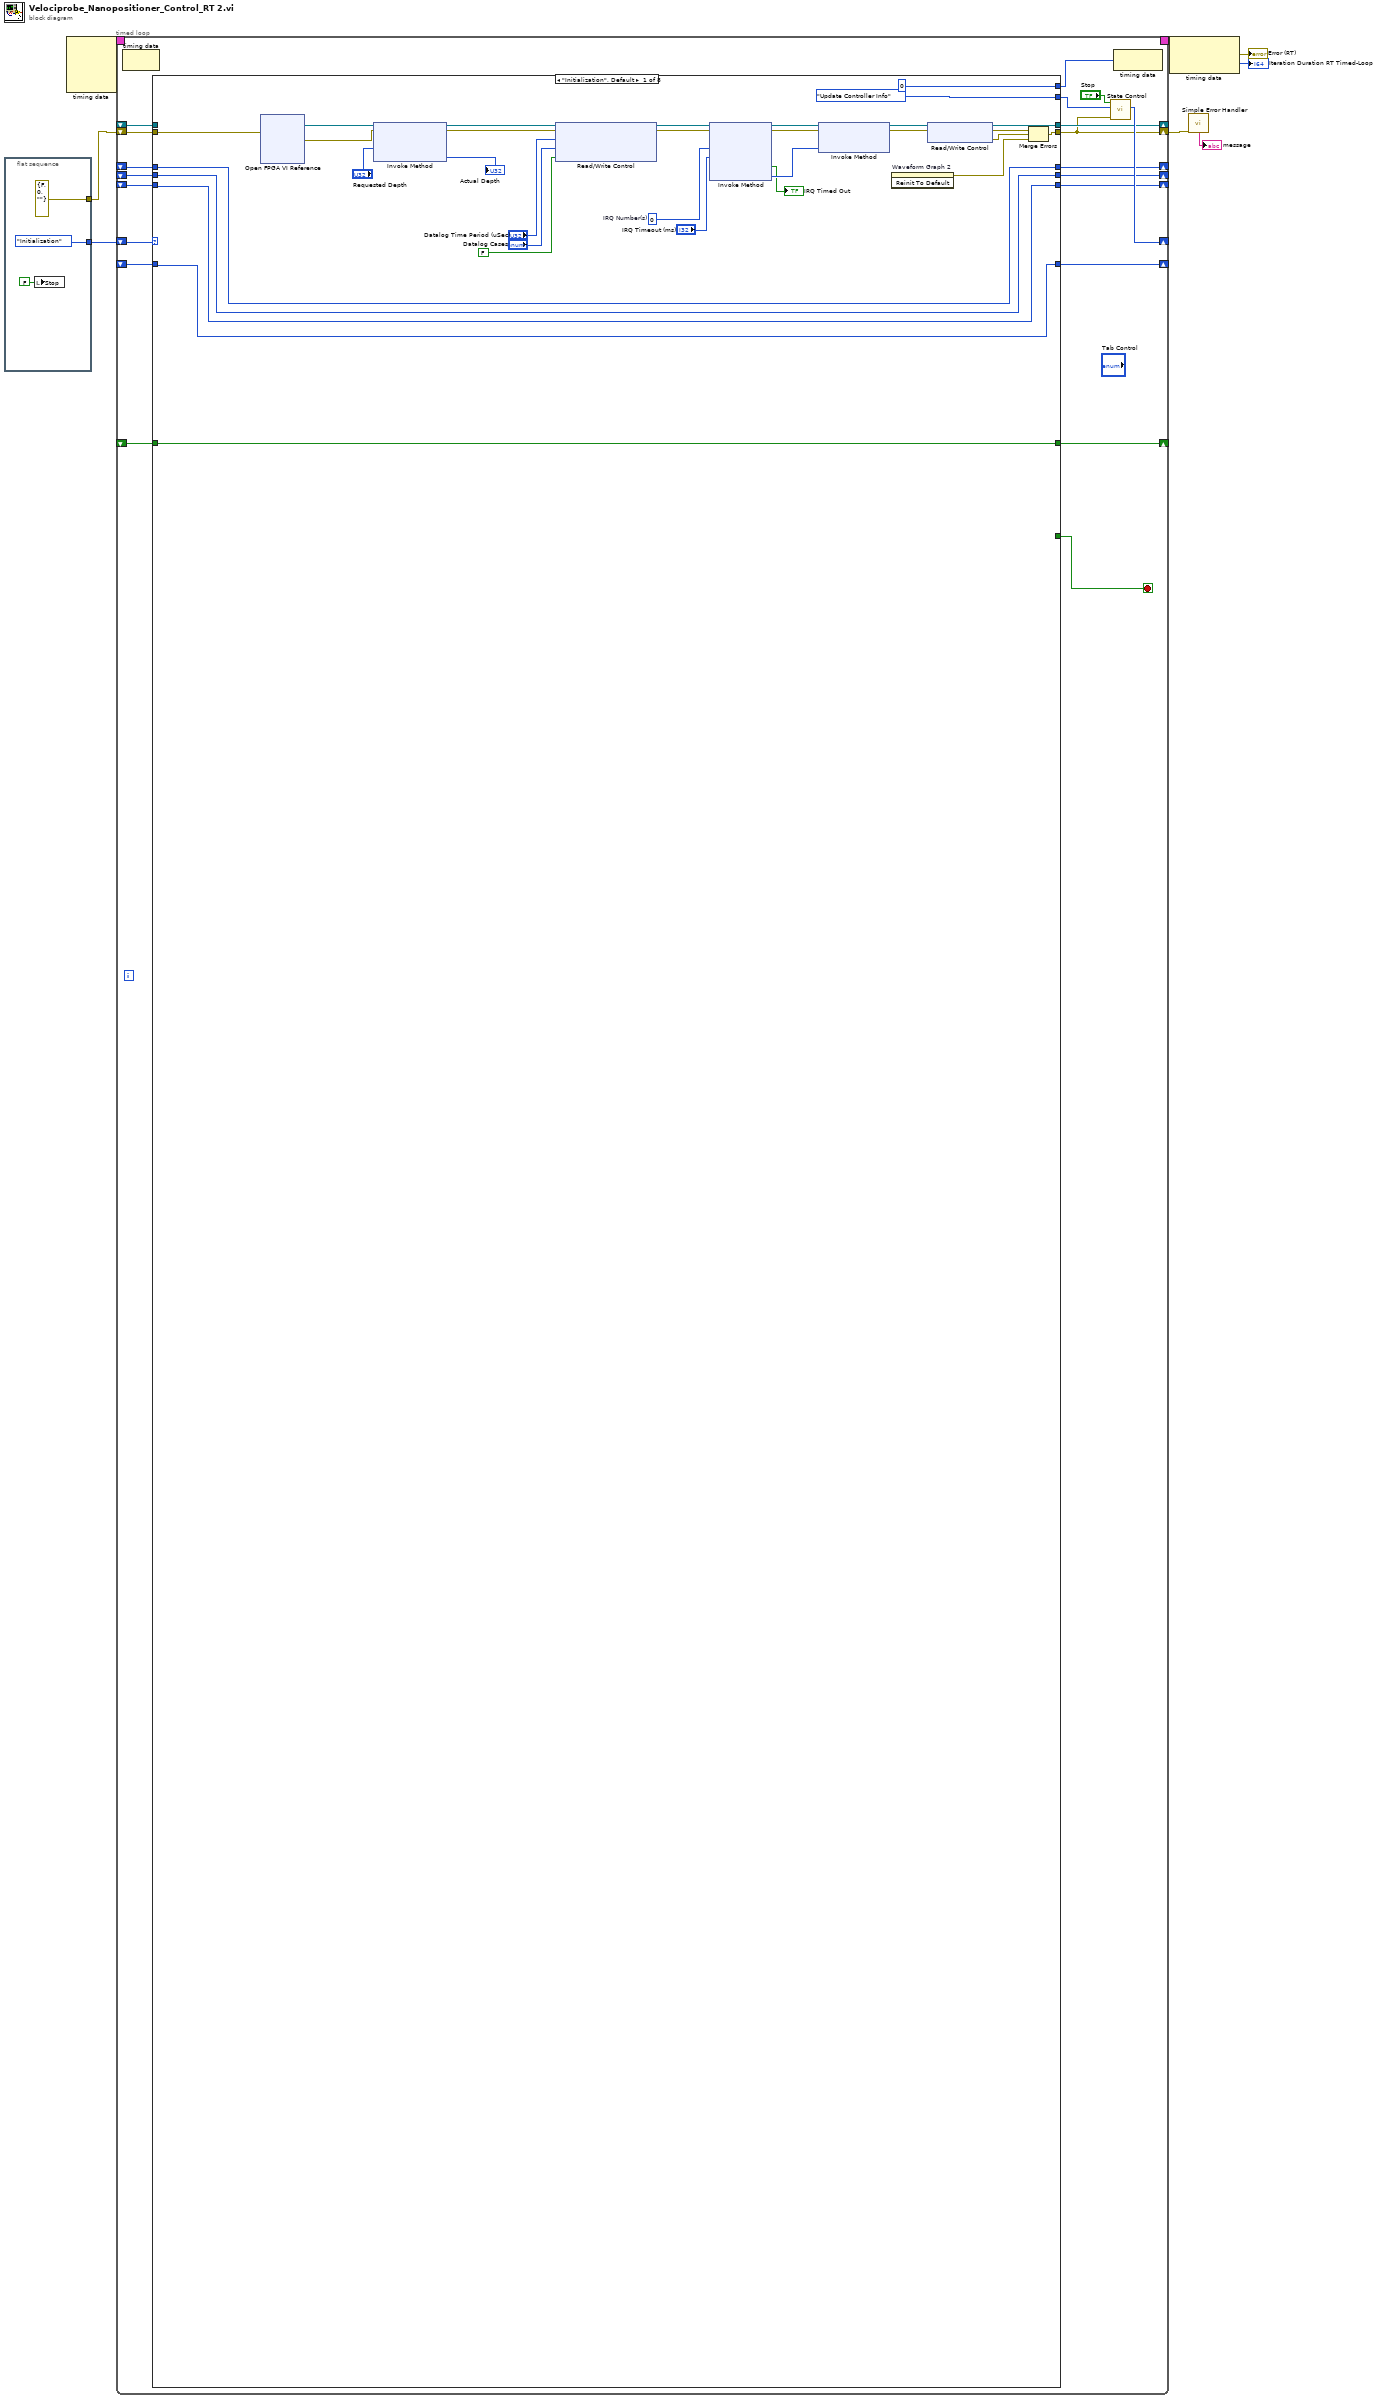
[diagram p0: block diagram]
diagram:
  n1 = flat-sequence {
    tunnel: [State_Enum."Initialization" ("States")] -> w6
    tunnel: [errorcluster {"status"=FALSE, "code"=0, "source"=""} ("error constant")] -> w2
    frame #0 {
      n2 = local write "Stop"(FALSE ("Stop")) -> ()
    }
  }
  n3 = node-c288() -> (w8:T9)  [unwired: 4 in]
  n4 = timed-loop {
    timing: w8 -> [_]
    timing-out: [_] -> w7
    shift-right: [w30] -> _
    shift-left: _ -> [w29]
    shift-right: [w24] -> _
    shift-left: w6 -> [w28]
    shift-right: [w23] -> _
    shift-left: _ -> [w22]
    shift-right: [w21] -> _
    shift-left: _ -> [w20]
    shift-right: [w18] -> _
    shift-left: _ -> [w19]
    shift-right: [w17] -> _
    shift-left: _ -> [w16]
    shift-right: [w15] -> _
    shift-left: _ -> [w12]
    shift-right: [w14] -> w1
    shift-left: w2 -> [w13]
    stop <- w27 stop-if-true
    n5 = node-c288() -> ()  [unwired: 1 in, 1 out]
    n6 = case shown="\"Initialization\", Default" w28 {
      tunnel: [i64 0 i64 0 i64 0 i64 0 i64 0 i64 0 i64 0 i64 0] -> w31
      tunnel: [w51 w64 w627 w728 w769 w803 w817 w899] -> w30
      tunnel: w29 -> [w51 w64 w627 w728 w769 w803 w851 w899]
      tunnel: [State_Enum."Update Controller Info" State_Enum."Update Reference Info" State_Enum."Update Detector Trigger Info" State_Enum."Update Datalog Info" ("States") State_Enum."Check FPGA Status" State_Enum."Reading FIFO" State_Enum."Update Controller Info" State_Enum."Initialization"] -> w25
      tunnel: [_ _ _ _ _ _ _ w900] -> w27
      tunnel: [w35 w74 w583 w723 w750 w802 w816 w898] -> w23
      tunnel: w22 -> [w35 w74 w582 w723 w750 w802 w816 w898]
      tunnel: [w34 w73 w579 w722 w749 w801 w815 w897] -> w21
      tunnel: w20 -> [w34 w73 w577 w722 w749 w801 w815 w897]
      tunnel: w19 -> [w33 w72 w574 w721 w748 w800 w814 w896]
      tunnel: [w33 w72 w578 w721 w748 w800 w814 w896] -> w18
      tunnel: [w32 w71 w569 w704 w747 w799 w828 w895] -> w17
      tunnel: w16 -> [w32 w71 w569 w703 w747 w799 w828 w895]
      tunnel: [w40 w66 w534 w695 w741 w796 w822 w890] -> w15
      tunnel: [w38 w65 w535 w694 w742 w794 w820 w888] -> w14
      tunnel: w13 -> [w37 w70 w538 w698 w745 w797 w825 w893]
      tunnel: w12 -> [_ w69 w539 w699 w746 w798 w826 w894]
      frame "Initialization", Default {
        w54 = 0  # IRQ Number(s)
        n7 = xnode ("Open FPGA VI Reference")("error in"=w37) -> ("FPGA VI Reference Out"=w36:refnum<k20>, "error out"=w49:errorcluster)  [unwired: 1 in]
        n8 = xnode "Invoke Method"("FPGA VI Reference In"=w36, "error in"=w49, "Requested Depth"="Requested Depth") -> ("FPGA VI Reference Out"=w48:refnum<k20>, "error out"=w47:errorcluster, "Actual Depth"=→"Actual Depth":u32)
        n9 = xnode "Read/Write Control"("FPGA VI Reference In"=w48, "error in"=w47, "Datalog Time Period (uSec)"="Datalog Time Period (uSec)", "Datalog Cases"="Datalog Cases", "Interrupt Boolean"=FALSE) -> ("FPGA VI Reference Out"=w46:refnum<k20>, "error out"=w45:errorcluster)
        n10 = xnode "Invoke Method"("FPGA VI Reference In"=w46, "error in"=w45, "IRQ Number(s)"=w54, "Timeout (ms)"="IRQ Timeout (ms)") -> ("FPGA VI Reference Out"=w44:refnum<k20>, "error out"=w43:errorcluster, "Timed Out"=→"IRQ Timed Out":bool, "IRQ(s) Asserted"=w56:i32)
        n11 = xnode "Invoke Method"("FPGA VI Reference In"=w44, "error in"=w43, "IRQ Number(s)"=w56) -> ("FPGA VI Reference Out"=w42:refnum<k20>, "error out"=w41:errorcluster)